vi "IMAQdx_AbsImage_Flea3_v4.6.vi"() -> ()   [LabVIEW 2013] (continued)
  out "Image note":string="Experiment=Sr\nCamera_ID=FL3_32S2M\nImageType=Raw\nDataType=Absorption\nImageDirection=XZ\nMagnification=1.000000E+0\nWMfreq=4.348288461E+2\nLastSave=8a4a9dcffc4e3239d56d97c71c6d4c8385ad02e2\nFileNumber=160\nIndex=0\nIndexedWaves=BBcaptureT;BBcompT;BlueLaserBeatnote;BlueLaserLockOffset;BlueLaserProbeBN;DipAOMFreq;DipPowCr;DipPowCr2;DipPowCr3;DipPowX;DipPowX2;DipPowX3;DipPowX4;DipPowZ;DipPowZ2;DipPowZ3;DipPowZLat;DoppCoolDet;DoppCoolStirDet;DoppCoolSweep;MOTPow;MOTPow2;MOTcurrent;Nspacers;Pdet;PixisPosition;ProbeDet;SFcoolT;TOF;TOFaux;WMfreq;Xshim;Yshim;ZShimVarF;Zshim;ZshimDC;ZshimVar;bLoadT;bMapT;bRampT;combWidthF;combWidthI;depumpOn;depumpPow;dopCoolT;evapOn;freq;holdT;loadT;pulseLatT;rMOTbroadDetuningF;rMOTbroadDetuningI;rMOTcurrF;rMOTcurrI;rMOTon;rMOTpow2;rMOTpow3;rMOTpow4;rMOTpow5;rMOTpow6;rMOTstirDetF;rMOTstirDetI;rampLatOffT;rampLatT;rampOn;rampT;singleFreqDet;singleFreqDetF;singleFreqStirDet;singleFreqStirDetF;tEvap1;tEvap2;tau;tau2;varWaveP1\nIndexedValues=50.0000000000000E-3;400.000000000000E-3;412.000000000000E+3;8.75000000000000E+0;419.000000000000E+3;40.2000000000000E+6;800.000000000000E-3;1.60000000000000E+0;30.0000000000000E-3;1.60000000000000E+0;3.20000000000000E+0;60.0000000000000E-3;30.0000000000000E-3;100.000000000000E-3;400.000000000000E-3;20.0000000000000E-3;150.000000000000E-3;-4.94000000000000E+3;-4.98000000000000E+3;-20.0000000000000E+0;10.0000000000000E+0;2.00000000000000E+0;-6.00000000000000E+0;4.00000000000000E+0;7.00000000000000E+0;15.3000000000000E+0;0.00000000000000E+0;10.0000000000000E-3;11.5000000000000E-3;10.0000000000000E-3;0.00000000000000E+0;230.000000000000E-3;2.55000000000000E+0;1.31500000000000E+0;1.75000000000000E+0;1.31500000000000E+0;1.31500000000000E+0;3.90000000000000E+0;400.000000000000E-6;75.0000000000000E-3;25.0000000000000E-3;2.00000000000000E+0;0.00000000000000E+0;1.00000000000000E+0;25.0000000000000E-3;1.00000000000000E+0;100.000000000000E+0;100.000000000000E-3;45.0000000000000E-3;3.00000000000000E-6;5.56000000000000E+0;5.56000000000000E+0;-290.000000000000E-3;-200.000000000000E-3;1.00000000000000E+0;1.70000000000000E+0;7.10000000000000E+0;1.90000000000000E+0;1.20000000000000E+0;1.65000000000000E+0;6.05000000000000E+0;6.05000000000000E+0;3.00000000000000E-3;50.0000000000000E-3;0.00000000000000E+0;200.000000000000E-3;-5.34000000000000E+3;-5.31000000000000E+3;-5.52000000000000E+3;-5.45000000000000E+3;3.20000000000000E+0;3.50000000000000E+0;1.00000000000000E+0;6.00000000000000E+0;2.65000000000000E+0\n# Current Variables\n#\nZShimVarF = 1.315000E+0\nZshimVar = 1.315000E+0\nBBcaptureT = 5.000000E-2\nBBcompT = 4.000000E-1\nBlueDipPow = 2.400000E-1\nBlueLaserBeatnote = 4.120000E+5\nBlueLaserLockOffset = 8.750000E+0\nBlueLaserProbeBN = 4.190000E+5\nDipAOMFreq = 4.020000E+7\nDipPowCr = 8.000000E-1\nDipPowCr2 = 1.600000E+0\nDipPowCr3 = 3.000000E-2\nDipPowCr4 = 1.500000E-2\nDipPowCrTOF = 8.000000E-1\nDipPowHLat = 7.700000E-2\nDipPowHLat2 = 4.500000E-1\nDipPowX = 1.600000E+0\nDipPowX2 = 3.200000E+0\nDipPowX3 = 6.000000E-2\nDipPowX4 = 3.000000E-2\nDipPowXLat = 1.000000E+0\nDipPowXTOF = 1.600000E+0\nDipPowZ = 1.000000E-1\nDipPowZ2 = 4.000000E-1\nDipPowZ3 = 2.000000E-2\nDipPowZ4 = 1.000000E-2\nDipPowZLat = 1.500000E-1\nDoppCoolDet = -4.940000E+3\nDoppCoolPow = 1.250000E+0\nDoppCoolStirDet = -4.980000E+3\nDoppCoolSweep = -2.000000E+1\nDoppStirPow = 1.600000E+0\nHeatingAmp = 1.000000E-1\nHimaging = 1.000000E+0\nMOTPow = 1.000000E+1\nMOTPow2 = 2.000000E+0\nMOTcurrent = -6.000000E+0\nMOTcurrent2 = -7.500000E+0\nMOTdetuning = -4.504000E+1\nNspacers = 4.000000E+0\nPdet = 7.000000E+0\nPdet2 = 5.000000E-2\nPixisPosition = 1.530000E+1\nProbeDet = 0.000000E+0\nProbePow = 1.420000E+0\nSFcoolT = 1.000000E-2\nTOF = 1.150000E-2\nTOFaux = 1.000000E-2\nVimaging = 1.000000E+0\nWMfreq = 0.000000E+0\nXshim = 2.300000E-1\nXshimDC = 2.500000E-1\nYshim = 2.550000E+0\nYshimDC = 2.575000E+0\nZshim = 1.750000E+0\nZshimDC = 1.315000E+0\nbLoadT = 3.900000E+0\nbMOToverride = 1.000000E+0\nbMapT = 4.000000E-4\nbRampT = 7.500000E-2\ncameraArmT = 1.500000E-3\ncombWidthF = 2.500000E-2\ncombWidthI = 2.000000E+0\ncompensation = -3.981000E+0\ndepumpOn = 0.000000E+0\ndepumpPow = 1.000000E+0\ndopCoolT = 2.500000E-2\ndopCoolT1 = 5.000000E-3\nevapOn = 1.000000E+0\nexposureT = 1.000000E-5\nfreq = 1.000000E+2\nholdT = 1.000000E-1\nloadT = 4.500000E-2\nminus_zman = -7.904000E+0\nplus_zman = -9.792000E+0\npulseLatT = 3.000000E-6\nrMOTbroadDetuningF = 5.560000E+0\nrMOTbroadDetuningI = 5.560000E+0\nrMOTcurrF = -2.900000E-1\nrMOTcurrI = -2.000000E-1\nrMOTon = 1.000000E+0\nrMOTpow1 = 7.000000E+0\nrMOTpow2 = 1.700000E+0\nrMOTpow3 = 7.100000E+0\nrMOTpow4 = 1.900000E+0\nrMOTpow5 = 1.200000E+0\nrMOTpow6 = 1.650000E+0\nrMOTstirDetF = 6.050000E+0\nrMOTstirDetI = 6.050000E+0\nrampLatOffT = 3.000000E-3\nrampLatT = 5.000000E-2\nrampOn = 0.000000E+0\nrampT = 2.000000E-1\nsingleFreqDet = -5.340000E+3\nsingleFreqDetF = -5.310000E+3\nsingleFreqStirDet = -5.520000E+3\nsingleFreqStirDetF = -5.450000E+3\nstirWidthF = 2.500000E-2\nstirWidthI = 2.000000E+0\ntEvap0 = 1.000000E-1\ntEvap1 = 3.200000E+0\ntEvap2 = 3.500000E+0\ntau = 1.000000E+0\ntau2 = 6.000000E+0\nvarWaveP1 = 2.650000E+0\nvarWaveP2 = 1.200000E+0\n#\n# Master Staging List\n#Comment\tMarker\tMode\tGroup\tDelay\tX ODT Shuttter\tX ODT AO TTL\tVert ODT Shutter\tVert ODT AO TTL\tCross ODT Shutter\tCross ODT AO TTL\t707 Shutter\tPB_7\tH Probe AO TTL\tFreq Switch rMOT\trMOT AO TTL\t\tTrans AO TTL\tV Probe AO TTL\tZman AO TTL\tbMOT AO TTL\t60 Hz Trig Gate\tWindow Heater TTL\tPB_18\t\tPB_20 Trigger Dev3\tPB_21 Trigger Dev2\tPB_22 Trigger Dev1\tPB_23 Trigger Dev0\tStep\t~Atomic Beam Shutter\tGate Valve\tDO0_2\t707b Shutter\t~Zman Coils\t~ MOT Coils\t~ Dipole Flea3 Shutter\trMOT Shutter\t+Zeeman Coils\t-Zeeman Coils\tCompensation Coils\tMOT Coils\trMOT AO Power\trMOT Freq Amplitude\trMOT Freq Offset\tH Lattice AO Power\tTrans Shutter\tV Probe Shutter\tZman Shutter\tbMOT Shutter\tDO1_4\t679 Shutter\t~Pixis Shutter\t~Abs Flea3 Shutter\tAO1_0\tMOT AO Power\tProbe AO Power\tAO1_3\tX Shim Coils\tY Shim Coils\tZ Shim Coils\tVert ODT AO Power\tPIXIS Ext Shutter\tBlueODT TTL\tBlueODT Shutter\tH Probe Shutter\tH Lattice Shutter\tH Lattice AO TTL\tParametric Heating\t689c AOM TTL\tAO2_0\tAO2_1\tD03_0\tD03_1\tD03_2\tD03_3\tD03_4\tD03_5\tD03_6\tD03_7\trMOT Stir Freq Offset\tBlueODT Power\tCrossODT Power\tVariable Waveplate\tAO3_4\tAO3_5\trMOT Stir Power\tX ODT AO Power\tSRS Freq\tSRS Amp\tSRS Offset\tSRS Func Type\tRedMotDDS\tRedMotDDS_ 0\tRedMotDDS_ 1\tRedMotDDS_ 2\tStirringDDS\tStirringDDS_ 0\tStirringDDS_ 1\tStirringDDS_ 2\tBlueBN\tBlueBN_ 0\tPosition\tRun Mode\r\n\r\nreset\t\tRamp\t1\t.1\t1\t1\t1\t1\t1\t1\t1\t0\t1\t0\t1\t0\t1\t1\t1\t0\t0\t0\t0\t0\t0\t0\t0\t0\t0\t0\t1\t0\t1\t0\t0\t1\t0\tplus_zman\tminus_zman\tcompensation\tMOTcurrent\trMOTpow1\tcombAmplitude(combWidthI)\trMOTdelta(-(rMOTbroadDetuningI +combWidthI/2))\tODTpowHLat(DipPowHLat2)\t0\t0\t1\t0\t0\t1\t1\t1\tbMOTdelta(MOTdetuning)\tbMOTpow(0.5)\tProbePow\tPdet2\tXshim\tYshim\tZshim\tODTpowZ(DipPowZ)\t0\t1\t0\t0\t0\t1\t0\t0\t0\t0\t0\t0\t0\t0\t0\t0\t0\t0\trMOTdelta(-(rMOTstirDetI +stirWidthI/2))\tODTpowBlue(0)\tODTpowXY(DipPowCr)\tvarWaveP1\tBlueLaserLockOffset\tAmp688(depumpPow)\trMOTpow3\tODTpowX(DipPowX)\tfreq\tHeatingAmp\t0\tSine\tDetuning\tsingleFreqDet\t-20\t8\tDetuning\tsingleFreqStirDet\t0\t0\tBlueBN\tBlueLaserBeatnote\tPixisPos(TOF)\tCycle Wait for Move\r\nblue MOT load\t\tRamp\t0\tbLoadT\t1\t1\t1\t1\t1\t1\t1\t0\t1\t0\t1\t0\t1\t1\t1\t1\t0\t0\t0\t0\t0\t0\t0\t0\t0\t0\t1\t0\t1\t0\t0\t1\t1\tplus_zman\tminus_zman\tcompensation\tMOTcurrent\trMOTpow1\tcombAmplitude(combWidthI)\trMOTdelta(-(rMOTbroadDetuningI +combWidthI/2))\tODTpowHLat(DipPowHLat)\t1\t0\t1\tbMOToverride\t1\t1\t1\t1\tbMOTdelta(MOTdetuning)\tbMOTpow(MOTPow)\tProbePow\tPdet2\tXshim\tYshim\tZshim\tODTpowZ(DipPowZ)\t0\t1\t0\t0\t0\t1\t0\t0\t0\t0\t0\t0\t0\t0\t0\t0\t0\t0\trMOTdelta(-(rMOTstirDetI +stirWidthI/2))\tODTpowBlue(0)\tODTpowXY(DipPowCr)\tvarWaveP1\tBlueLaserLockOffset\tAmp688(depumpPow)\trMOTpow3\tODTpowX(DipPowX)\tfreq\tHeatingAmp\t0\tSine\tDetuning\tsingleFreqDet\t-20\t8\tDetuning\tsingleFreqStirDet\t0\t0\tBlueBN\tBlueLaserBeatnote\tPixisPos(TOF)\tCycle Wait for Move\r\npretrig\t\tRamp\t1\t500m\t1\t1\t1\t1\t1\t0\t1\t0\t1\t0\t1\t0\t1\t1\t1\t1\t0\t1\t0\t0\t0\t0\t0\t0\t0\t0\t1\t0\t1\t0\t0\t0\t1\tplus_zman\tminus_zman\tcompensation\tMOTcurrent\trMOTpow1\tcombAmplitude(combWidthI)\trMOTdelta(-(rMOTbroadDetuningI +combWidthI/2))\tODTpowHLat(DipPowHLat2)\t1\t0\t1\tbMOToverride\t1\t1\t0\t0\tbMOTdelta(MOTdetuning)\tbMOTpow(MOTPow)\tProbePow\tPdet2\tXshim\tYshim\tZshim\tODTpowZ(DipPowZ)\t0\t1\t0\t0\t1\t1\t0\t0\t0\t0\t0\t0\t0\t0\t0\t0\t0\t0\trMOTdelta(-(rMOTstirDetI +stirWidthI/2))\tODTpowBlue(0)\tODTpowXY(DipPowCr)\tvarWaveP1\tBlueLaserLockOffset\tAmp688(depumpPow)\trMOTpow3\tODTpowX(DipPowX)\tfreq\tHeatingAmp\t0\tSine\tDetuning\tsingleFreqDet\t-20\t8\tDetuning\tsingleFreqStirDet\t0\t0\tBlueBN\tBlueLaserBeatnote\tPixisPos(TOF)\tCycle Wait for Move\r\nblue MOT load\t\tRamp\t1\tbLoadT\t1\t1\t1\t1\t1\t1\t1\t0\t1\t0\t1\t0\t1\t1\t1\t1\t0\t0\t0\t0\t0\t0\t0\t0\t0\t0\t1\t0\t1\t0\t0\t1\t1\tplus_zman\tminus_zman\tcompensation\tMOTcurrent\trMOTpow1\tcombAmplitude(combWidthI)\trMOTdelta(-(rMOTbroadDetuningI +combWidthI/2))\tODTpowHLat(DipPowHLat)\t1\t0\t1\tbMOToverride\t1\t1\t1\t1\tbMOTdelta(MOTdetuning)\tbMOTpow(MOTPow)\tProbePow\tPdet2\tXshim\tYshim\tZshim\tODTpowZ(DipPowZ)\t0\t1\t0\t0\t0\t1\t0\t0\t0\t0\t0\t0\t0\t0\t0\t0\t0\t0\trMOTdelta(-(rMOTstirDetI +stirWidthI/2))\tODTpowBlue(0)\tODTpowXY(DipPowCr)\tvarWaveP1\tBlueLaserLockOffset\tAmp688(depumpPow)\trMOTpow3\tODTpowX(DipPowX)\tfreq\tHeatingAmp\t0\tSine\tDetuning\tsingleFreqDet\t-20\t8\tDetuning\tsingleFreqStirDet\t0\t0\tBlueBN\tBlueLaserBeatnote\tPixisPos(TOF)\tCycle Wait for Move\r\ndump bMOT\t\tRamp\t1\t0.1-bRampT\t1\t1\t1\t1\t1\t1\t1\t0\t1\t0\t1\t0\t1\t1\t1\t1\t0\t1\t0\t0\t0\t0\t0\t0\t1m\t0\t1\t0\t1\t0\t0\t1\t1\tplus_zman\tminus_zman\tcompensation\tMOTcurrent\trMOTpow1\tcombAmplitude(combWidthI)\trMOTdelta(-(rMOTbroadDetuningI +combWidthI/2))\tODTpowHLat(DipPowHLat)\t1\t0\t1\tbMOToverride\t1\t1\t1\t1\tbMOTdelta(MOTdetuning)\tbMOTpow(MOTPow)\tProbePow\tPdet2\tXshim\tYshim\tZshim\tODTpowZ(DipPowZ)\t0\t1\t0\t0\t0\t1\t0\t0\t0\t0\t0\t0\t0\t0\t0\t0\t0\t0\trMOTdelta(-(rMOTstirDetI +stirWidthI/2))\tODTpowBlue(0)\tODTpowXY(DipPowCr)\tvarWaveP1\tBlueLaserLockOffset\tAmp688(depumpPow)\trMOTpow3\tODTpowX(DipPowX)\tfreq\tHeatingAmp\t0\tSine\tDetuning\tsingleFreqDet\t-20\t8\tDetuning\tsingleFreqStirDet\t0\t0\tBlueBN\tBlueLaserBeatnote\tPixisPos(TOF)\tCycle Wait for Move\r\ndump bMOT\t\tRamp\t1\tbRampT\t1\t1\t1\t1\t1\t1\t1\t0\t1\t0\t1\t0\t1\t1\t1\t1\t0\t1\t0\t0\t0\t0\t0\t0\t1m\t0\t1\t0\t1\t0\t0\t1\t1\tplus_zman\tminus_zman\tcompensation\tLineRamp(f,MOTcurrent,MOTcurrent2)\trMOTpow1\tcombAmplitude(combWidthI)\trMOTdelta(-(rMOTbroadDetuningI +combWidthI/2))\tODTpowHLat(DipPowHLat)\t1\t0\t1\tbMOToverride\t1\t1\t1\t1\tbMOTdelta(MOTdetuning)\tLineRamp(f,bMOTpow(MOTPow),bMOTpow(MOTPow2))\tProbePow\tPdet2\tXshim\tYshim\tZshim\tODTpowZ(DipPowZ)\t0\t1\t0\t0\t0\t1\t0\t0\t0\t0\t0\t0\t0\t0\t0\t0\t0\t0\trMOTdelta(-(rMOTstirDetI +stirWidthI/2))\tODTpowBlue(0)\tODTpowXY(DipPowCr)\tvarWaveP1\tBlueLaserLockOffset\tAmp688(depumpPow)\trMOTpow3\tODTpowX(DipPowX)\tfreq\tHeatingAmp\t0\tSine\tDetuning\tsingleFreqDet\t-20\t8\tDetuning\tsingleFreqStirDet\t0\t0\tBlueBN\tBlueLaserBeatnote\tPixisPos(TOF)\tCycle Wait for Move\r\nCamWaitTime\t\tRamp\t0\t.1\t1\t1\t1\t1\t1\t1\t1\t0\t0\t0\t1\t0\t1\t0\t1\t1\t0\t1\t0\t0\t0\t0\t0\t0\t0\t0\t1\t0\t1\t0\t0\t1\t1\tplus_zman\tminus_zman\tcompensation\tMOTcurrent\trMOTpow1\tcombAmplitude(combWidthI)\trMOTdelta(-(rMOTbroadDetuningI +combWidthI/2))\tODTpowHLat(DipPowHLat)\t1\t0\t1\tbMOToverride\t1\t1\t1\t1\tbMOTdelta(MOTdetuning)\tbMOTpow(MOTPow2)\tProbePow\tPdet2\tXshim\tYshim\tZshim\tODTpowZ(DipPowZ)\t0\t1\t0\t0\t0\t1\t0\t0\t0\t0\t0\t0\t0\t0\t0\t0\t0\t0\trMOTdelta(-(rMOTstirDetI +stirWidthI/2))\tODTpowBlue(0)\tODTpowXY(DipPowCr)\tvarWaveP1\tBlueLaserLockOffset\tAmp688(depumpPow)\trMOTpow3\tODTpowX(DipPowX)\tfreq\tHeatingAmp\t0\tSine\tDetuning\tsingleFreqDet\t-20\t8\tDetuning\tsingleFreqStirDet\t0\t0\tBlueBN\tBlueLaserBeatnote\tPixisPos(TOF)\tCycle Wait for Move\r\nProbeShutOn\t\tRamp\t1-rMOTon\t1120e-6\t1\t1\t1\t1\t1\t1\t1\t0\t0\t0\t1\t0\t0\t0\t0\t1\t0\t1\t0\t0\t0\t0\t0\t0\t0\t0\t1\t0\t1\t0\t0\t1\t1\tplus_zman\tminus_zman\tcompensation\tMOTcurrent\trMOTpow1\tcombAmplitude(combWidthI)\trMOTdelta(-(rMOTbroadDetuningI +combWidthI/2))\tODTpowHLat(DipPowHLat)\t1\t0\t1\tbMOToverride\t1\t1\t1\t1\tbMOTdelta(MOTdetuning)\tbMOTpow(MOTPow2)\tProbePow\tPdet2\tXshim\tYshim\tZshim\tODTpowZ(DipPowZ)\t0\t1\t0\tHimaging\t0\t1\t0\t0\t0\t0\t0\t0\t0\t0\t0\t0\t0\t0\trMOTdelta(-(rMOTstirDetI +stirWidthI/2))\tODTpowBlue(0)\tODTpowXY(DipPowCr)\tvarWaveP1\tBlueLaserLockOffset\tAmp688(depumpPow)\trMOTpow3\tODTpowX(DipPowX)\tfreq\tHeatingAmp\t0\tSine\tDetuning\tsingleFreqDet\t-20\t8\tDetuning\tsingleFreqStirDet\t0\t0\tBlueBN\tBlueLaserBeatnote\tPixisPos(TOF)\tCycle Wait for Move\r\nRepumpShutOff\t\tRamp\t1-rMOTon\t260e-6\t1\t1\t1\t1\t1\t1\t1\t0\t0\t0\t1\t0\t0\t0\t0\t1\t0\t1\t0\t0\t0\t0\t0\t0\t0\t0\t1\t0\t1\t0\t0\t1\t1\tplus_zman\tminus_zman\tcompensation\tMOTcurrent\trMOTpow1\tcombAmplitude(combWidthI)\trMOTdelta(-(rMOTbroadDetuningI +combWidthI/2))\tODTpowHLat(DipPowHLat)\t1\t0\t0\tbMOToverride\t1\t1\t1\t1\tbMOTdelta(MOTdetuning)\tbMOTpow(MOTPow2)\tProbePow\tPdet2\tXshim\tYshim\tZshim\tODTpowZ(DipPowZ)\t0\t1\t0\tHimaging\t0\t1\t0\t0\t0\t0\t0\t0\t0\t0\t0\t0\t0\t0\trMOTdelta(-(rMOTstirDetI +stirWidthI/2))\tODTpowBlue(0)\tODTpowXY(DipPowCr)\tvarWaveP1\tBlueLaserLockOffset\tAmp688(depumpPow)\trMOTpow3\tODTpowX(DipPowX)\tfreq\tHeatingAmp\t0\tSine\tDetuning\tsingleFreqDet\t-20\t8\tDetuning\tsingleFreqStirDet\t0\t0\tBlueBN\tBlueLaserBeatnote\tPixisPos(TOF)\tCycle Wait for Move\r\nMOTShutOff\t\tRamp\t1-rMOTon\t1370e-6\t1\t1\t1\t1\t1\t1\t1\t0\t0\t0\t1\t0\t0\t0\t0\t1\t0\t1\t0\t0\t0\t0\t0\t0\t0\t0\t1\t0\t1\t0\t0\t1\t1\tplus_zman\tminus_zman\tcompensation\tMOTcurrent\trMOTpow1\tcombAmplitude(combWidthI)\trMOTdelta(-(rMOTbroadDetuningI +combWidthI/2))\tODTpowHLat(DipPowHLat)\t1\t0\t0\t0\t1\t1\t1\t1\tbMOTdelta(MOTdetuning)\tbMOTpow(MOTPow2)\tProbePow\tPdet2\tXshim\tYshim\tZshim\tODTpowZ(DipPowZ)\t0\t1\t0\tHimaging\t0\t1\t0\t0\t0\t0\t0\t0\t0\t0\t0\t0\t0\t0\trMOTdelta(-(rMOTstirDetI +stirWidthI/2))\tODTpowBlue(0)\tODTpowXY(DipPowCr)\tvarWaveP1\tBlueLaserLockOffset\tAmp688(depumpPow)\trMOTpow3\tODTpowX(DipPowX)\tfreq\tHeatingAmp\t0\tSine\tDetuning\tsingleFreqDet\t-20\t8\tDetuning\tsingleFreqStirDet\t0\t0\tBlueBN\tBlueLaserBeatnote\tPixisPos(TOF)\tCycle Wait for Move\r\nCoil Switch\t\tRamp\trMOTon\t220e-6\t1\t1\t1\t1\t1\t1\t1\t0\t1\t0\t1\t0\t0\t1\t0\t1\t0\t1\t0\t0\t0\t0\t0\t0\t0\t0\t1\t0\t1\t0\t0\t1\t1\tplus_zman\tminus_zman\tcompensation\trMOTcurrI\trMOTpow1\tcombAmplitude(combWidthI)\trMOTdelta(-(rMOTbroadDetuningI +combWidthI/2))\tODTpowHLat(DipPowHLat)\t1\t0\t0\t0\t1\t1\t1\t1\tbMOTdelta(MOTdetuning)\tbMOTpow(2)\tProbePow\tPdet2\tXshim\tYshim\tZshim\tODTpowZ(DipPowZ)\t0\t1\t0\t0\t0\t1\t0\t0\t0\t0\t0\t0\t0\t0\t0\t0\t0\t0\trMOTdelta(-(rMOTstirDetI +stirWidthI/2))\tODTpowBlue(0)\tODTpowXY(DipPowCr)\tvarWaveP1\tBlueLaserLockOffset\tAmp688(depumpPow)\trMOTpow3\tODTpowX(DipPowX)\tfreq\tHeatingAmp\t0\tSine\tDetuning\tsingleFreqDet\t-20\t8\tDetuning\tsingleFreqStirDet\t0\t0\tBlueBN\tBlueLaserBeatnote\tPixisPos(TOF)\tCycle Wait for Move\r\n60HzTrigger\t\tHalt\t0\t10u\t1\t1\t1\t1\t1\t1\t1\t0\t0\t0\t1\t0\t0\t0\t0\t0\t0\t1\t0\t0\t0\t0\t0\t0\t0\t0\t1\t0\t1\t0\t0\t1\t1\tplus_zman\tminus_zman\tcompensation\trMOTcurrI\trMOTpow1\tcombAmplitude(combWidthI)\trMOTdelta(-(rMOTbroadDetuningI +combWidthI/2))\tODTpowHLat(DipPowHLat)\t1\t0\t0\t0\t1\t1\t1\t1\tbMOTdelta(MOTdetuning)\tbMOTpow(2)\tProbePow\tPdet2\tXshim\tYshim\tZshim\tODTpowZ(DipPowZ)\t0\t1\t0\t0\t0\t1\t0\t0\t0\t0\t0\t0\t0\t0\t0\t0\t0\t0\trMOTdelta(-(rMOTstirDetI +stirWidthI/2))\tODTpowBlue(0)\tODTpowXY(DipPowCr)\tvarWaveP1\tBlueLaserLockOffset\tAmp688(depumpPow)\trMOTpow3\tODTpowX(DipPowX)\tfreq\tHeatingAmp\t0\tSine\tDetuning\tsingleFreqDet\t-20\t8\tDetuning\tsingleFreqStirDet\t0\t0\tBlueBN\tBlueLaserBeatnote\tPixisPos(TOF)\tCycle Wait for Move\r\nCapture Red MOT\t\tRamp\trMOTon\tBBcaptureT\t1\t1\t1\t1\t1\t1\t1\t0\t1\t0\t1\t0\t0\t1\t0\t0\t0\t1\t0\t0\t0\t0\t0\t0\t1m\t0\t1\t0\t1\t0\t0\t1\t1\tplus_zman\tminus_zman\tcompensation\trMOTcurrI\trMOTpow1\tcombAmplitude(combWidthI)\trMOTdelta(-(rMOTbroadDetuningI +combWidthI/2))\tODTpowHLat(DipPowHLat)\t0\t0\t0\t0\t1\t1\t1\t1\tbMOTdelta(MOTdetuning)\tbMOTpow(0.5)\tProbePow\tPdet2\tXshim\tYshim\tZshim\tODTpowZ(DipPowZ)\t0\t1\t0\t0\t0\t1\t0\t0\t0\t0\t0\t0\t0\t0\t0\t0\t0\t0\trMOTdelta(-(rMOTstirDetI +stirWidthI/2))\tODTpowBlue(0)\tODTpowXY(DipPowCr)\tvarWaveP1\tBlueLaserLockOffset\tAmp688(depumpPow)\trMOTpow3\tODTpowX(DipPowX)\tfreq\tHeatingAmp\t0\tSine\tDetuning\tsingleFreqDet\t-20\t8\tDetuning\tsingleFreqStirDet\t0\t0\tBlueBN\tBlueLaserProbeBN\tPixisPos(TOF)\tCycle Wait for Move\r\nRamp Red MOT\t\tRamp\trMOTon\tBBcompT\t1\t1\t1\t1\t1\t1\t1\t0\t1\t0\t1\t0\t0\t1\t0\t0\t0\t1\t0\t0\t0\t0\t0\t0\t10u\t0\t1\t0\t1\t0\t0\t1\t1\tplus_zman\tminus_zman\tcompensation\tLineRamp(f,rMOTcurrI,rMOTcurrF)\tHalfGaussRamp(t,rMOTpow1,rMOTpow2, BBcompT)\tLineRamp(f,combAmplitude(combWidthI),combAmplitude(combWidthF))\tLineRamp(f,rMOTdelta(-(rMOTbroadDetuningI +combWidthI/2)),rMOTdelta(-(rMOTbroadDetuningF +combWidthF/2)))\tODTpowHLat(DipPowHLat)\t0\t0\t0\t0\t1\t1\t1\t1\tbMOTdelta(MOTdetuning)\tbMOTpow(0.5)\tProbePow\tPdet2\tXshim\tYshim\tLineRamp(f,Zshim,ZshimVar)\tODTpowZ(DipPowZ)\t0\t1\t0\t0\t0\t1\t0\t0\t0\t0\t0\t0\t0\t0\t0\t0\t0\t0\tLineRamp(f,rMOTdelta(-(rMOTstirDetI +stirWidthI/2)),rMOTdelta(-(rMOTstirDetF +stirWidthF/2)))\tODTpowBlue(0)\tODTpowXY(DipPowCr)\tvarWaveP1\tLineRamp(f,BlueLaserLockOffset,Pdet)\tAmp688(depumpPow)\tHalfGaussRamp(t,rMOTpow3,rMOTpow4, BBcompT)\tODTpowX(DipPowX)\tfreq\tHeatingAmp\t0\tSine\tDetuning\tsingleFreqDet\t-20\t8\tDetuning\tsingleFreqStirDet\t0\t0\tBlueBN\tBlueLaserProbeBN\tPixisPos(TOF)\tCycle Wait for Move\r\nBB load\t\tRamp\t0\tloadT\t1\t1\t1\t1\t1\t1\t0\t0\t0\t0\t1\t0\t0\t0\t0\t0\t0\t1\t0\t0\t0\t0\t0\t0\t10u\t0\t1\t0\t0\t0\t0\t1\t1\tplus_zman\tminus_zman\tcompensation\trMOTcurrF\trMOTpow2\tcombAmplitude(combWidthF)\trMOTdelta(-(rMOTbroadDetuningF +combWidthF/2))\tODTpowHLat(DipPowHLat)\t0\t0\t0\t0\t1\t0\t1\t1\tbMOTdelta(MOTdetuning)\tbMOTpow(0.5)\tProbePow\tPdet2\tXshim\tYshim\tLineRamp(f,ZshimVar,ZShimVarF)\tODTpowZ(DipPowZ)\t0\t1\t0\t0\t0\t1\t0\t0\t0\t0\t0\t0\t0\t0\t0\t0\t0\t0\trMOTdelta(-(rMOTstirDetF +stirWidthF/2))\tODTpowBlue(0)\tODTpowXY(DipPowCr)\tvarWaveP1\tPdet\tAmp688(depumpPow)\trMOTpow4\tODTpowX(DipPowX)\tfreq\tHeatingAmp\t0\tSine\tDetuning\tsingleFreqDet\t-20\t8\tDetuning\tsingleFreqStirDet\t0\t0\tBlueBN\tBlueLaserProbeBN\tPixisPos(TOF)\tCycle Wait for Move\r\nSF\t\tRamp\t1\tSFcoolT\t1\t1\t1\t1\t1\t1\t0\t0\t0\t1\t1\t0\t0\t0\t0\t0\t0\t1\t0\t0\t0\t0\t0\t0\t10u\t0\t1\t0\t0\t0\t0\t1\t1\tplus_zman\tminus_zman\tcompensation\trMOTcurrF\trMOTpow2\tcombAmplitude(combWidthF)\trMOTdelta(-(rMOTbroadDetuningF +combWidthF/2))\tODTpowHLat(DipPowHLat)\t0\t0\t0\t0\t1\t0\t1\t1\tbMOTdelta(MOTdetuning)\tbMOTpow(0.5)\tProbePow\tPdet2\tXshim\tYshim\tZshimVar\tODTpowZ(DipPowZ)\t0\t1\t0\t0\t0\t1\t0\t0\t0\t0\t0\t0\t0\t0\t0\t0\t0\t0\trMOTdelta(-(rMOTstirDetF +stirWidthF/2))\tODTpowBlue(0)\tODTpowXY(DipPowCr)\tvarWaveP1\tPdet\tAmp688(depumpPow)\trMOTpow4\tODTpowX(DipPowX)\tfreq\tHeatingAmp\t0\tSine\tRamp\tsingleFreqDet\tsingleFreqDet + 20\tSFCoolT*1000\tRamp\tsingleFreqStirDet\tsingleFreqStirDet + 20\tSFcoolT*1000\tBlueBN\tBlueLaserProbeBN\tPixisPos(TOF)\tCycle Wait for Move\r\nload1\t\tRamp\t1\tloadT\t1\t1\t1\t1\t1\t1\t1\t0\t1\t1\t1\t0\t0\t1\t0\t0\t0\t1\t0\t0\t0\t0\t0\t0\t10u\t0\t1\t0\t0\t0\t0\t1\t1\tplus_zman\tminus_zman\tcompensation\trMOTcurrF\tLineRamp(f,rMOTpow2,rMOTpow5)\tcombAmplitude(combWidthF)\trMOTdelta(-(rMOTbroadDetuningF +combWidthF/2))\tODTpowHLat(DipPowHLat)\t0\t0\t0\t0\t1\t0\t1\t1\tbMOTdelta(MOTdetuning)\tbMOTpow(0.5)\tProbePow\tPdet2\tXshim\tYshim\tLineRamp(f,ZshimVar,ZShimVarF)\tODTpowZ(DipPowZ)\t0\t1\t0\t0\t0\t1\t0\t0\t0\t0\t0\t0\t0\t0\t0\t0\t0\t0\trMOTdelta(-(rMOTstirDetF +stirWidthF/2))\tODTpowBlue(0)\tODTpowXY(DipPowCr)\tvarWaveP1\tPdet\tAmp688(depumpPow)\tLineRamp(f,rMOTpow4,rMOTpow6)\tODTpowX(DipPowX)\tfreq\tHeatingAmp\t0\tSine\tDetuning\tsingleFreqDetF\tsingleFreqDet + 20\tSFCoolT*1000\tDetuning\tsingleFreqStirDet + 20\tsingleFreqStirDet + 20\tSFcoolT*1000\tBlueBN\tBlueLaserProbeBN\tPixisPos(TOF)\tCycle Wait for Move\r\nload2\t\tRamp\t0\t.05\t1\t1\t1\t1\t1\t1\t0\t0\t1\t1\t1\t0\t0\t1\t0\t0\t0\t1\t0\t0\t0\t0\t0\t0\t0\t0\t1\t0\t0\t0\t0\t1\t1\tplus_zman\tminus_zman\tcompensation\trMOTcurrF\trMOTpow5\tcombAmplitude(combWidthF)\trMOTdelta(-(rMOTbroadDetuningF +combWidthF/2))\tODTpowHLat(DipPowHLat)\t0\t0\t0\t0\t1\t0\t1\t1\tbMOTdelta(MOTdetuning)\tbMOTpow(0.5)\tProbePow\tPdet2\tXshim\tYshim\tZshimVar\tODTpowZ(DipPowZ)\t0\t1\t0\t0\t0\t1\t0\t0\t0\t0\t0\t0\t0\t0\t0\t0\t0\t0\trMOTdelta(-(rMOTstirDetF +stirWidthF/2))\tODTpowBlue(0)\tODTpowXY(DipPowCr)\tvarWaveP1\tPdet\tAmp688(depumpPow)\trMOTpow6\tODTpowX(DipPowX)\tfreq\tHeatingAmp\t0\tSine\tDetuning\tsingleFreqDetF\tsingleFreqDet + 20\tSFCoolT*1000\tDetuning\tsingleFreqStirDetF\tsingleFreqStirDet + 20\tSFcoolT*1000\tBlueBN\tBlueLaserProbeBN\tPixisPos(TOF)\tCycle Wait for Move\r\ndrop Red MOT\t\tRamp\t0\t.15\t1\t1\t0\t0\t0\t0\t0\t0\t1\t1\t0\t0\t0\t1\t0\t0\t0\t1\t0\t0\t0\t0\t0\t0\t0\t0\t1\t0\t0\t0\t1\t1\t0\tplus_zman\tminus_zman\tcompensation\trMOTcurrF\trMOTpow5\tcombAmplitude(combWidthF)\trMOTdelta(-(rMOTbroadDetuningF +combWidthF/2))\tODTpowHLat(DipPowHLat2)\t0\t0\t0\t0\t0\t0\t1\t1\tbMOTdelta(MOTdetuning)\tbMOTpow(0.5)\tProbePow\tPdet2\tXshim\tYshim\tZShimVarF\tODTpowZ(DipPowZ)\t0\t1\t0\t0\t1\t1\t0\t0\t0\t0\t0\t0\t0\t0\t0\t0\t0\t0\trMOTdelta(-(rMOTstirDetF +stirWidthF/2))\tODTpowBlue(0)\tODTpowXY(DipPowCr)\tvarWaveP1\tPdet\tAmp688(depumpPow)\trMOTpow6\tODTpowX(DipPowX)\tfreq\tHeatingAmp\t0\tSine\tDetuning\tDoppCoolDet\tsingleFreqDet + 20\tSFCoolT*1000\tDetuning\tDoppCoolStirDet\tsingleFreqStirDet + 20\tSFcoolT*1000\tBlueBN\tBlueLaserProbeBN\tPixisPos(TOF)\tCycle Wait for Move\r\nramp Trap\t\tRamp\t1\trampT\t1\t1\t1\t1\t1\t1\t0\t0\t1\t1\t0\t0\t0\t1\t0\t0\t0\t1\t0\t0\t0\t0\t0\t0\t10u\t0\t1\t0\t0\t0\t1\t1\t0\tplus_zman\tminus_zman\tcompensation\trMOTcurrF\trMOTpow3\tcombAmplitude(combWidthF)\trMOTdelta(-(rMOTbroadDetuningF +combWidthF/2))\tODTpowHLat(DipPowHLat)\t0\t0\t0\t0\t0\t0\t1\t1\tbMOTdelta(MOTdetuning)\tbMOTpow(0.5)\tProbePow\tPdet2\tXshimDC\tYshimDC\tZshimDC\tSinRamp(t,(ODTpowZ(DipPowZ)+ODTpowZ(DipPowZ2))/2,(ODTpowZ(DipPowZ2)-ODTpowZ(DipPowZ))/2,1/(2*rampT),3*pi/2)\t0\t1\t0\t0\t0\t1\t0\t0\t0\t0\t0\t0\t0\t0\t0\t0\t0\t0\trMOTdelta(-(rMOTstirDetI +stirWidthF/2))\tODTpowBlue(0)\tSinRamp(t,(ODTpowXY(DipPowCr)+ODTpowXY(DipPowCr2))/2,(ODTpowXY(DipPowCr2)-ODTpowXY(DipPowCr))/2,1/(2*rampT),3*pi/2)\tvarWaveP1\tPdet\tAmp688(depumpPow)\trMOTpow6\tSinRamp(t,(ODTpowX(DipPowX)+ODTpowX(DipPowX2))/2,(ODTpowX(DipPowX2)-ODTpowX(DipPowX))/2,1/(2*rampT),3*pi/2)\tfreq\tHeatingAmp\t0\tSine\tDetuning\tsingleFreqDetF\tsingleFreqDet + 20\tSFCoolT*1000\tDetuning\tsingleFreqStirDetF\tsingleFreqStirDet + 20\tSFcoolT*1000\tBlueBN\tBlueLaserProbeBN\tPixisPos(TOF)\tCycle Wait for Move\r\nhold\t\tRamp\t0\t.01\t1\t1\t1\t1\t1\t1\t0\t0\t1\t1\t0\t0\t0\t1\t0\t0\t0\t1\t0\t0\t0\t0\t0\t0\t0\t0\t1\t0\t0\t0\t1\t1\t0\tplus_zman\tminus_zman\tcompensation\trMOTcurrF\trMOTpow4\tcombAmplitude(combWidthF)\trMOTdelta(-(rMOTbroadDetuningF +combWidthF/2))\tODTpowHLat(DipPowHLat)\t0\t0\t0\t0\t1\t0\t1\t1\tbMOTdelta(MOTdetuning)\tbMOTpow(0.5)\tProbePow\tPdet2\tXshimDC\tYshimDC\tZshimDC\tODTpowZ(DipPowZ2)\t0\t1\t0\t0\t0\t1\t0\t0\t0\t0\t0\t0\t0\t0\t0\t0\t0\t0\trMOTdelta(-(rMOTstirDetI +stirWidthF/2))\tODTpowBlue(0)\tODTpowXY(DipPowCr2)\tvarWaveP1\tPdet\tAmp688(depumpPow)\trMOTpow6\tODTpowX(DipPowX2)\tfreq\tHeatingAmp\t0\tSine\tDetuning\tDoppCoolDetF\tsingleFreqDet + 20\tSFCoolT*1000\tDetuning\tDoppCoolStirDet\tsingleFreqStirDet + 20\tSFcoolT*1000\tBlueBN\tBlueLaserProbeBN\tPixisPos(TOF)\tCycle Wait for Move\r\nramp Trap\t\tRamp\t0\trampT\t1\t1\t1\t1\t1\t1\t0\t0\t1\t1\t0\t0\t0\t1\t0\t0\t0\t1\t0\t0\t0\t0\t0\t0\t10u\t0\t1\t0\t0\t0\t1\t1\t0\tplus_zman\tminus_zman\tcompensation\trMOTcurrF\trMOTpow3\tcombAmplitude(combWidthF)\trMOTdelta(-(rMOTbroadDetuningF +combWidthF/2))\tODTpowHLat(DipPowHLat)\t0\t0\t0\t0\t0\t0\t1\t1\tbMOTdelta(MOTdetuning)\tbMOTpow(0.5)\tProbePow\tPdet2\tXshimDC\tYshimDC\tZshimDC\tSinRamp(t,(ODTpowZ(DipPowZ)+ODTpowZ(DipPowZ2))/2,(ODTpowZ(DipPowZ2)-ODTpowZ(DipPowZ))/2,1/(2*rampT),pi/2)\t0\t1\t0\t0\t0\t1\t0\t0\t0\t0\t0\t0\t0\t0\t0\t0\t0\t0\trMOTdelta(-(rMOTstirDetI +stirWidthF/2))\tODTpowBlue(0)\tSinRamp(t,(ODTpowXY(DipPowCr)+ODTpowXY(DipPowCr2))/2,(ODTpowXY(DipPowCr2)-ODTpowXY(DipPowCr))/2,1/(2*rampT),pi/2)\tvarWaveP1\tPdet\tAmp688(depumpPow)\trMOTpow6\tSinRamp(t,(ODTpowX(DipPowX)+ODTpowX(DipPowX2))/2,(ODTpowX(DipPowX2)-ODTpowX(DipPowX))/2,1/(2*rampT),pi/2)\tfreq\tHeatingAmp\t0\tSine\tDetuning\tsingleFreqDetF\tsingleFreqDet + 20\tSFCoolT*1000\tDetuning\tsingleFreqStirDetF\tsingleFreqStirDet + 20\tSFcoolT*1000\tBlueBN\tBlueLaserProbeBN\tPixisPos(TOF)\tCycle Wait for Move\r\nhold\t\tRamp\t0\t.5\t1\t1\t1\t1\t1\t1\t0\t0\t1\t1\t0\t0\t0\t1\t0\t0\t0\t1\t0\t0\t0\t0\t0\t0\t0\t0\t1\t0\t0\t0\t1\t1\t0\tplus_zman\tminus_zman\tcompensation\trMOTcurrF\trMOTpow4\tcombAmplitude(combWidthF)\trMOTdelta(-(rMOTbroadDetuningF +combWidthF/2))\tODTpowHLat(DipPowHLat)\t0\t0\t0\t0\t1\t0\t1\t1\tbMOTdelta(MOTdetuning)\tbMOTpow(0.5)\tProbePow\tPdet2\tXshimDC\tYshimDC\tZshimDC\tODTpowZ(DipPowZ)\t0\t1\t0\t0\t0\t1\t0\t0\t0\t0\t0\t0\t0\t0\t0\t0\t0\t0\trMOTdelta(-(rMOTstirDetI +stirWidthF/2))\tODTpowBlue(0)\tODTpowXY(DipPowCr)\tvarWaveP1\tPdet\tAmp688(depumpPow)\trMOTpow6\tODTpowX(DipPowX)\tfreq\tHeatingAmp\t0\tSine\tDetuning\tDoppCoolDetF\tsingleFreqDet + 20\tSFCoolT*1000\tDetuning\tDoppCoolStirDet\tsingleFreqStirDet + 20\tSFcoolT*1000\tBlueBN\tBlueLaserProbeBN\tPixisPos(TOF)\tCycle Wait for Move\r\nDoppler Cool1\t\tRamp\t0\tdopCoolT\t1\t1\t1\t1\t1\t1\t0\t0\t1\t1\t1\t0\t0\t1\t0\t0\t0\t1\t0\t0\t0\t0\t0\t0\t10u\t0\t1\t0\t0\t0\t1\t1\t1\tplus_zman\tminus_zman\tcompensation\trMOTcurrF\tDoppCoolPow\tcombAmplitude(combWidthF)\trMOTdelta(-(rMOTbroadDetuningF +combWidthF/2))\tODTpowHLat(DipPowHLat)\t0\t0\t0\t0\t1\t0\t1\t1\tbMOTdelta(MOTdetuning)\tbMOTpow(0.5)\tProbePow\tPdet2\tXshimDC\tYshimDC\tZshimDC\tODTpowZ(DipPowZ)\t0\t1\t0\t0\t0\t1\t0\t0\t0\t0\t0\t0\t0\t0\t0\t0\t0\t0\trMOTdelta(-(rMOTstirDetI +stirWidthF/2))\tODTpowBlue(0)\tODTpowXY(DipPowCr)\tvarWaveP1\tPdet\tAmp688(depumpPow)\tDoppStirPow\tODTpowX(DipPowX2)\tfreq\tHeatingAmp\t0\tSine\tDetuning\tDoppCoolDet\tsingleFreqDet + 20\tSFCoolT*1000\tDetuning\tDoppCoolStirDet\tsingleFreqStirDet + 20\tSFcoolT*1000\tBlueBN\tBlueLaserProbeBN\tPixisPos(TOF)\tCycle Wait for Move\r\nDoppler Cool2\t\tRamp\t0\tdopCoolT\t1\t1\t1\t1\t1\t1\t0\t0\t1\t1\t1\t0\t0\t1\t0\t0\t0\t1\t0\t0\t0\t0\t0\t0\t10u\t0\t1\t0\t0\t0\t1\t1\t1\tplus_zman\tminus_zman\tcompensation\trMOTcurrF\trMOTpow5\tcombAmplitude(combWidthF)\trMOTdelta(-(rMOTbroadDetuningF +combWidthF/2))\tODTpowHLat(DipPowHLat)\t0\t0\t0\t0\t1\t0\t1\t1\tbMOTdelta(MOTdetuning)\tbMOTpow(0.5)\tProbePow\tPdet2\tXshimDC\tYshimDC\tZshimDC\tODTpowZ(DipPowZ)\t0\t1\t0\t0\t0\t1\t0\t0\t0\t0\t0\t0\t0\t0\t0\t0\t0\t0\trMOTdelta(-(rMOTstirDetI +stirWidthF/2))\tODTpowBlue(0)\tODTpowXY(DipPowCr)\tvarWaveP1\tPdet\tAmp688(depumpPow)\trMOTpow6\tODTpowX(DipPowX2)\tfreq\tHeatingAmp\t0\tSine\tRamp\tDoppCoolDet\tDoppCoolDet-DoppCoolSweep\tdopCoolT*1000\tDetuning\tDoppCoolStirDet\tsingleFreqStirDet + 20\tSFcoolT*1000\tBlueBN\tBlueLaserProbeBN\tPixisPos(TOF)\tCycle Wait for Move\r\nDoppler Cool3\t\tRamp\t0\tdopCoolT\t1\t1\t1\t1\t1\t1\t0\t0\t1\t1\t1\t0\t0\t1\t0\t0\t0\t1\t0\t0\t0\t0\t0\t0\t10u\t0\t1\t0\t0\t0\t1\t1\t1\tplus_zman\tminus_zman\tcompensation\trMOTcurrF\tLineRamp(f,rMOTpow4,rMOTpow5)\tcombAmplitude(combWidthF)\trMOTdelta(-(rMOTbroadDetuningF +combWidthF/2))\tODTpowHLat(DipPowHLat)\t0\t0\t0\t0\t1\t0\t1\t1\tbMOTdelta(MOTdetuning)\tbMOTpow(0.5)\tProbePow\tPdet2\tXshimDC\tYshimDC\tZshimDC\tODTpowZ(DipPowZ)\t0\t1\t0\t0\t0\t1\t0\t0\t0\t0\t0\t0\t0\t0\t0\t0\t0\t0\trMOTdelta(-(rMOTstirDetI +stirWidthF/2))\tODTpowBlue(0)\tODTpowXY(DipPowCr)\tvarWaveP1\tPdet\tAmp688(depumpPow)\tLineRamp(f,rMOTpow4,rMOTpow5)\tODTpowX(DipPowX2)\tfreq\tHeatingAmp\t0\tSine\tDetuning\tDoppCoolDet-DoppCoolSweep\tDoppCoolDet-DoppCoolSweep\tdopCoolT*1000\tDetuning\tDoppCoolStirDet\tsingleFreqStirDet + 20\tSFcoolT*1000\tBlueBN\tBlueLaserProbeBN\tPixisPos(TOF)\tCycle Wait for Move\r\nhold\t\tRamp\t0\t2\t1\t1\t0\t0\t0\t0\t0\t0\t1\t1\t0\t0\t0\t1\t0\t0\t0\t1\t0\t0\t0\t0\t0\t0\t0\t0\t1\t0\t0\t0\t1\t1\t0\tplus_zman\tminus_zman\tcompensation\trMOTcurrF\trMOTpow4\tcombAmplitude(combWidthF)\trMOTdelta(-(rMOTbroadDetuningF +combWidthF/2))\tODTpowHLat(DipPowHLat)\t0\t0\t0\t0\t0\t0\t1\t1\tbMOTdelta(MOTdetuning)\tbMOTpow(0.5)\tProbePow\tPdet2\tXshim\tYshim\tZshimVar\tODTpowZ(DipPowZ)\t0\t1\t0\t0\t0\t1\t0\t0\t0\t0\t0\t0\t0\t0\t0\t0\t0\t0\trMOTdelta(-(rMOTstirDetI +stirWidthF/2))\tODTpowBlue(0)\tODTpowXY(DipPowCr2)\tvarWaveP1\tPdet\tAmp688(depumpPow)\trMOTpow4\tLineRamp(f, ODTpowX(DipPowX), ODTpowX(DipPowX2))\tfreq\tHeatingAmp\t0\tSine\tDetuning\tDoppCoolDet-DoppCoolSweep\tDoppCoolDet-DoppCoolSweep\tdopCoolT*1000\tDetuning\tDoppCoolStirDet\tsingleFreqStirDet + 20\tSFcoolT*1000\tBlueBN\tBlueLaserProbeBN\tPixisPos(TOF)\tCycle Wait for Move\r\nhold\t\tRamp\t0\tholdT\t1\t1\t0\t0\t0\t0\t0\t0\t1\t1\t0\t0\t0\t1\t0\t0\t0\t1\t0\t0\t0\t0\t0\t0\t0\t0\t1\t0\t0\t0\t1\t1\t0\tplus_zman\tminus_zman\tcompensation\trMOTcurrF\trMOTpow4\tcombAmplitude(combWidthF)\trMOTdelta(-(rMOTbroadDetuningF +combWidthF/2))\tODTpowHLat(DipPowHLat2)\t0\t0\t0\t0\t0\t0\t1\t1\tbMOTdelta(MOTdetuning)\tbMOTpow(0.5)\tProbePow\tPdet2\tXshim\tYshim\tZshimVar\tODTpowZ(DipPowZ)\t0\t1\t0\t0\t1\t1\t0\t0\t0\t0\t0\t0\t0\t0\t0\t0\t0\t0\trMOTdelta(-(rMOTstirDetI +stirWidthF/2))\tODTpowBlue(0)\tODTpowXY(DipPowCr)\tvarWaveP1\tPdet\tAmp688(depumpPow)\trMOTpow4\tODTpowX(DipPowX)\tfreq\tHeatingAmp\t0\tSine\tDetuning\tDoppCoolDet-DoppCoolSweep\tDoppCoolDet-DoppCoolSweep\tdopCoolT*1000\tDetuning\tDoppCoolStirDet\tsingleFreqStirDet + 20\tSFcoolT*1000\tBlueBN\tBlueLaserProbeBN\tPixisPos(TOF)\tCycle Wait for Move\r\ndrop HTrap\t\tRamp\t0\t.03\t1\t1\t1\t1\t1\t1\t0\t0\t1\t1\t0\t0\t0\t1\t0\t0\t0\t1\t0\t0\t0\t0\t0\t0\t0\t0\t1\t0\t0\t0\t1\t1\t0\tplus_zman\tminus_zman\tcompensation\trMOTcurrF\trMOTpow3\tcombAmplitude(combWidthF)\trMOTdelta(-(rMOTbroadDetuningF +combWidthF/2))\tODTpowHLat(DipPowHLat)\t0\t0\t0\t0\t0\t0\t1\t1\tbMOTdelta(MOTdetuning)\tbMOTpow(0.5)\tProbePow\tPdet2\tXshim\tYshim\tZshimVar\tODTpowZ(DipPowZ)\t0\t1\t0\t0\t0\t1\t0\t0\t0\t0\t0\t0\t0\t0\t0\t0\t0\t0\trMOTdelta(-(rMOTstirDetI +stirWidthF/2))\tODTpowBlue(0)\tODTpowXY(DipPowCr)\tvarWaveP1\tPdet\tAmp688(depumpPow)\trMOTpow3\tODTpowX(DipPowX)\tfreq\tHeatingAmp\t0\tSine\tDetuning\tsingleFreqDet\tDoppCoolDet-DoppCoolSweep\tdopCoolT*1000\tDetuning\tsingleFreqStirDet + 20\tsingleFreqStirDet + 20\tSFcoolT*1000\tBlueBN\tBlueLaserProbeBN\tPixisPos(TOF)\tCycle Wait for Move\r\nmodulate\t\tRamp\t0\t3m\t1\t1\t1\t1\t1\t1\t0\t0\t1\t1\t0\t0\t0\t1\t0\t0\t0\t1\t0\t0\t0\t0\t0\t0\t0\t0\t1\t0\t0\t0\t1\t1\t0\tplus_zman\tminus_zman\tcompensation\trMOTcurrF\trMOTpow3\tcombAmplitude(combWidthF)\trMOTdelta(-(rMOTbroadDetuningF +combWidthF/2))\tODTpowHLat(DipPowHLat)\t0\t0\t0\t0\t0\t0\t1\t1\tbMOTdelta(MOTdetuning)\tbMOTpow(0.5)\tProbePow\tPdet2\tXshim\tYshim\tZshimVar\tODTpowZ(DipPowZ)\t0\t1\t0\t0\t0\t1\t0\t0\t0\t0\t0\t0\t0\t0\t0\t0\t0\t0\trMOTdelta(-(rMOTstirDetI +stirWidthF/2))\tODTpowBlue(0)\tODTpowXY(DipPowCr)\tvarWaveP1\tPdet\tAmp688(depumpPow)\trMOTpow3\tODTpowX(DipPowX)\tfreq\tHeatingAmp\t0\tSine\tDetuning\tsingleFreqDet\tDoppCoolDet-DoppCoolSweep\tdopCoolT*1000\tDetuning\tsingleFreqStirDet + 20\tsingleFreqStirDet + 20\tSFcoolT*1000\tBlueBN\tBlueLaserProbeBN\tPixisPos(TOF)\tCycle Wait for Move\r\nEvaporation\t\tRamp\tevapOn\ttEvap1\t1\t1\t1\t1\t1\t1\t0\t0\t1\t1\t0\t0\t0\t1\t0\t0\t0\t1\t0\t0\t0\t0\t0\t0\t1m\t0\t1\t0\t0\t0\t1\t1\t0\tplus_zman\tminus_zman\tcompensation\trMOTcurrF\trMOTpow3\tcombAmplitude(combWidthF)\trMOTdelta(-(rMOTbroadDetuningF +combWidthF/2))\tODTpowHLat(DipPowHLat)\t0\t0\t0\t0\t0\t0\t1\t1\tbMOTdelta(MOTdetuning)\tbMOTpow(0.5)\tProbePow\tPdet2\tXshim\tYshim\tZshimVar\tLineRamp(f,ODTpowZ(DipPowZ2),ODTpowZ(DipPowZ3))\t0\t1\t0\t0\t0\t1\t0\t0\t0\t0\t0\t0\t0\t0\t0\t0\t0\t0\trMOTdelta(-(rMOTstirDetI +stirWidthF/2))\tODTpowBlue(0)\tExpRamp2(t,0,ODTpowXY(DipPowCr2),ODTpowXY(DipPowCr3),tau)\tvarWaveP1\tPdet\tAmp688(depumpPow)\trMOTpow3\tExpRamp2(t,0,ODTpowX(DipPowX2),ODTpowX(DipPowX3),tau)\tfreq\tHeatingAmp\t0\tSine\tDetuning\tsingleFreqDet\tDoppCoolDet-DoppCoolSweep\tdopCoolT*1000\tDetuning\tsingleFreqStirDet + 20\tsingleFreqStirDet + 20\tSFcoolT*1000\tBlueBN\tBlueLaserProbeBN\tPixisPos(TOF)\tCycle Wait for Move\r\nlattice ramp\t\tRamp\t0\t10m\t1\t1\t1\t0\t1\t1\t0\t0\t1\t1\t0\t0\t0\t1\t0\t0\t0\t1\t0\t0\t0\t0\t0\t0\t0\t0\t1\t0\t0\t0\t1\t1\t0\tplus_zman\tminus_zman\tcompensation\trMOTcurrF\trMOTpow3\tcombAmplitude(combWidthF)\trMOTdelta(-(rMOTbroadDetuningF +combWidthF/2))\tODTpowHLat(DipPowHLat)\t0\t0\t0\t0\t0\t0\t1\t1\tbMOTdelta(MOTdetuning)\tbMOTpow(0.5)\tProbePow\tPdet2\tXshim\tYshim\tZshimVar\tODTpowZ(DipPowZ3)\t0\t1\t0\t0\t1\t0\t0\t0\t0\t0\t0\t0\t0\t0\t0\t0\t0\t0\trMOTdelta(-(rMOTstirDetI +stirWidthF/2))\tODTpowBlue(BlueDipPow)\tExpFinal(tEvap1,ODTpowXY(DipPowCr2),ODTpowXY(DipPowCr3),tau)\tvarWaveP2\tPdet\tAmp688(depumpPow)\trMOTpow3\tExpFinal(tEvap1,ODTpowX(DipPowX2),ODTpowX(DipPowX3),tau)\tfreq\tHeatingAmp\t0\tSine\tDetuning\tsingleFreqDet\tDoppCoolDet-DoppCoolSweep\tdopCoolT*1000\tDetuning\tsingleFreqStirDet + 20\tsingleFreqStirDet + 20\tSFcoolT*1000\tBlueBN\tBlueLaserProbeBN\tPixisPos(TOF)\tCycle Wait for Move\r\nbox ramp up\t\tRamp\t0\t1\t1\t1\t1\t1\t1\t1\t0\t0\t1\t1\t0\t0\t0\t1\t0\t0\t0\t1\t0\t0\t0\t0\t0\t0\t10m\t0\t1\t0\t0\t0\t1\t1\t0\tplus_zman\tminus_zman\tcompensation\trMOTcurrF\trMOTpow3\tcombAmplitude(combWidthF)\trMOTdelta(-(rMOTbroadDetuningF +combWidthF/2))\tODTpowHLat(DipPowHLat)\t0\t0\t0\t0\t0\t0\t1\t1\tbMOTdelta(MOTdetuning)\tbMOTpow(0.5)\tProbePow\tPdet2\tXshim\tYshim\tZshimVar\tODTpowZ(DipPowZ3)\t0\t1\t0\t0\t1\t0\t0\t0\t0\t0\t0\t0\t0\t0\t0\t0\t0\t0\trMOTdelta(-(rMOTstirDetI +stirWidthF/2))\tSinRamp(t,(ODTpowBlue(BlueDipPow)+ODTpowBlue(0))/2,(ODTpowBlue(BlueDipPow)-ODTpowBlue(0))/2,1/(2*1),3*pi/2)\tExpFinal(tEvap1,ODTpowXY(DipPowCr2),ODTpowXY(DipPowCr3),tau)\tvarWaveP1\tPdet\tAmp688(depumpPow)\trMOTpow3\tExpFinal(tEvap1,ODTpowX(DipPowX2),ODTpowX(DipPowX3),tau)\tfreq\tHeatingAmp\t0\tSine\tDetuning\tsingleFreqDet\tDoppCoolDet-DoppCoolSweep\tdopCoolT*1000\tDetuning\tsingleFreqStirDet + 20\tsingleFreqStirDet + 20\tSFcoolT*1000\tBlueBN\tBlueLaserProbeBN\tPixisPos(TOF)\tCycle Wait for Move\r\npost evap hold\t\tRamp\t1\t20m\t1\t1\t1\t1\t1\t1\t0\t0\t1\t1\t0\t0\t0\t1\t0\t0\t0\t1\t0\t0\t0\t0\t0\t0\t0\t0\t1\t0\t0\t0\t1\t1\t0\tplus_zman\tminus_zman\tcompensation\trMOTcurrF\trMOTpow3\tcombAmplitude(combWidthF)\trMOTdelta(-(rMOTbroadDetuningF +combWidthF/2))\tODTpowHLat(DipPowHLat2)\t0\t0\t0\t0\t0\t0\t1\t1\tbMOTdelta(MOTdetuning)\tbMOTpow(0.5)\tProbePow\tPdet2\tXshim\tYshim\tZshimVar\tODTpowZ(DipPowZ3)\t0\t1\t0\t0\t1\t0\t0\t0\t0\t0\t0\t0\t0\t0\t0\t0\t0\t0\trMOTdelta(-(rMOTstirDetI +stirWidthF/2))\tODTpowBlue(BlueDipPow)\tExpFinal(tEvap1,ODTpowXY(DipPowCr2),ODTpowXY(DipPowCr3),tau)\tvarWaveP1\tPdet\tAmp688(depumpPow)\trMOTpow3\tExpFinal(tEvap1,ODTpowX(DipPowX2),ODTpowX(DipPowX3),tau)\tfreq\tHeatingAmp\t0\tSine\tDetuning\tsingleFreqDet\tDoppCoolDet-DoppCoolSweep\tdopCoolT*1000\tDetuning\tsingleFreqStirDet + 20\tsingleFreqStirDet + 20\tSFcoolT*1000\tBlueBN\tBlueLaserProbeBN\tPixisPos(TOF)\tCycle Wait for Move\r\npost evap\t\tRamp\t1\tpulseLatT\t1\t1\t1\t1\t1\t1\t0\t0\t1\t1\t0\t0\t0\t1\t0\t0\t0\t1\t0\t0\t0\t0\t0\t0\t0\t0\t1\t0\t0\t0\t1\t1\t0\tplus_zman\tminus_zman\tcompensation\trMOTcurrF\trMOTpow3\tcombAmplitude(combWidthF)\trMOTdelta(-(rMOTbroadDetuningF +combWidthF/2))\tODTpowHLat(DipPowHLat2)\t0\t0\t0\t0\t0\t0\t1\t1\tbMOTdelta(MOTdetuning)\tbMOTpow(0.5)\tProbePow\tPdet2\tXshim\tYshim\tZshimVar\tODTpowZ(DipPowZ3)\t0\t1\t0\t0\t1\t1\t0\t0\t0\t0\t0\t0\t0\t0\t0\t0\t0\t0\trMOTdelta(-(rMOTstirDetI +stirWidthF/2))\tODTpowBlue(BlueDipPow)\tExpFinal(tEvap1,ODTpowXY(DipPowCr2),ODTpowXY(DipPowCr3),tau)\tvarWaveP1\tPdet\tAmp688(depumpPow)\trMOTpow3\tExpFinal(tEvap1,ODTpowX(DipPowX2),ODTpowX(DipPowX3),tau)\tfreq\tHeatingAmp\t0\tSine\tDetuning\tsingleFreqDet\tDoppCoolDet-DoppCoolSweep\tdopCoolT*1000\tDetuning\tsingleFreqStirDet + 20\tsingleFreqStirDet + 20\tSFcoolT*1000\tBlueBN\tBlueLaserProbeBN\tPixisPos(TOF)\tCycle Wait for Move\r\npost evap hold\t\tRamp\t0\t2*rampLatT\t1\t1\t1\t1\t1\t1\t0\t0\t1\t1\t0\t0\t0\t1\t0\t0\t0\t1\t0\t0\t0\t0\t0\t0\t0\t0\t1\t0\t0\t0\t1\t1\t0\tplus_zman\tminus_zman\tcompensation\trMOTcurrF\trMOTpow3\tcombAmplitude(combWidthF)\trMOTdelta(-(rMOTbroadDetuningF +combWidthF/2))\tODTpowHLat(DipPowHLat)\t0\t0\t0\t0\t0\t0\t1\t1\tbMOTdelta(MOTdetuning)\tbMOTpow(0.5)\tProbePow\tPdet2\tXshim\tYshim\tZshimVar\tODTpowZ(DipPowZ3)\t0\t1\t0\t0\t1\t0\t0\t0\t0\t0\t0\t0\t0\t0\t0\t0\t0\t0\trMOTdelta(-(rMOTstirDetI +stirWidthF/2))\tODTpowBlue(BlueDipPow)\tExpFinal(tEvap1,ODTpowXY(DipPowCr2),ODTpowXY(DipPowCr3),tau)\tvarWaveP1\tPdet\tAmp688(depumpPow)\trMOTpow3\tExpFinal(tEvap1,ODTpowX(DipPowX2),ODTpowX(DipPowX3),tau)\tfreq\tHeatingAmp\t0\tSine\tDetuning\tsingleFreqDet\tDoppCoolDet-DoppCoolSweep\tdopCoolT*1000\tDetuning\tsingleFreqStirDet + 20\tsingleFreqStirDet + 20\tSFcoolT*1000\tBlueBN\tBlueLaserProbeBN\tPixisPos(TOF)\tCycle Wait for Move\r\nlattice rampup\t\tRamp\t0\trampLatT\t1\t1\t1\t1\t1\t1\t0\t0\t1\t1\t0\t0\t0\t1\t0\t0\t0\t1\t0\t0\t0\t0\t0\t0\t10u\t0\t1\t0\t0\t0\t1\t1\t0\tplus_zman\tminus_zman\tcompensation\trMOTcurrF\trMOTpow3\tcombAmplitude(combWidthF)\trMOTdelta(-(rMOTbroadDetuningF +combWidthF/2))\tSinRamp(t,(ODTpowHLat(DipPowHLat)+ODTpowHLat(DipPowHLat2))/2,(ODTpowHLat(DipPowHLat)-ODTpowHLat(DipPowHLat2))/2,1/(2*rampLatT), pi/2)\t0\t0\t0\t0\t0\t0\t1\t1\tbMOTdelta(MOTdetuning)\tbMOTpow(0.5)\tProbePow\tPdet2\tXshim\tYshim\tZshimVar\tSinRamp(t,(ODTpowZ(DipPowZ3)+ODTpowZ(DipPowZLat))/2, (ODTpowZ(DipPowZ3)-ODTpowZ(DipPowZLat))/2, 1/(2*rampLatT), pi/2)\t0\t1\t0\t0\t1\t0\t0\t0\t0\t0\t0\t0\t0\t0\t0\t0\t0\t0\trMOTdelta(-(rMOTstirDetI +stirWidthF/2))\tODTpowBlue(0)\tExpFinal(tEvap1,ODTpowXY(DipPowCr2),ODTpowXY(DipPowCr3),tau)\tLineRamp(f,varWaveP1,varWaveP2)\tPdet\tAmp688(depumpPow)\trMOTpow3\tExpFinal(tEvap1,ODTpowX(DipPowX2),ODTpowX(DipPowX3),tau)\tfreq\tHeatingAmp\t0\tSine\tDetuning\tsingleFreqDet\tDoppCoolDet-DoppCoolSweep\tdopCoolT*1000\tDetuning\tsingleFreqStirDet + 20\tsingleFreqStirDet + 20\tSFcoolT*1000\tBlueBN\tBlueLaserProbeBN\tPixisPos(TOF)\tCycle Wait for Move\r\nODT rampdown\t\tRamp\t0\trampLatT\t1\t1\t1\t1\t1\t1\t0\t0\t1\t1\t0\t0\t0\t1\t0\t0\t0\t1\t0\t0\t0\t0\t0\t0\t1m\t0\t1\t0\t0\t0\t1\t1\t0\tplus_zman\tminus_zman\tcompensation\trMOTcurrF\trMOTpow3\tcombAmplitude(combWidthF)\trMOTdelta(-(rMOTbroadDetuningF +combWidthF/2))\tODTpowHLat(DipPowHLat2)\t0\t0\t0\t0\t0\t0\t1\t1\tbMOTdelta(MOTdetuning)\tbMOTpow(0.5)\tProbePow\tPdet2\tXshim\tYshim\tZshimVar\tODTpowZ(DipPowZLat)\t0\t1\t0\t0\t1\t1\t0\t0\t0\t0\t0\t0\t0\t0\t0\t0\t0\t0\trMOTdelta(-(rMOTstirDetI +stirWidthF/2))\tODTpowBlue(0)\tSinRamp(t,(ExpFinal(tEvap1,ODTpowXY(DipPowCr2),ODTpowXY(DipPowCr3),tau)+ODTpowXY(0))/2,(ODTpowXY(0)-ExpFinal(tEvap1,ODTpowXY(DipPowCr2),ODTpowXY(DipPowCr3),tau))/2,1/(2*rampLatT),3*pi/2)\tvarWaveP2\tPdet\tAmp688(depumpPow)\trMOTpow3\tSinRamp(t,(ExpFinal(tEvap1,ODTpowX(DipPowX2),ODTpowX(DipPowX3),tau)+ODTpowX(0))/2,(ODTpowX(0)-ExpFinal(tEvap1,ODTpowX(DipPowX2),ODTpowX(DipPowX3),tau))/2,1/(2*rampLatT),3*pi/2)\tfreq\tHeatingAmp\t0\tSine\tDetuning\tsingleFreqDet\tDoppCoolDet-DoppCoolSweep\tdopCoolT*1000\tDetuning\tsingleFreqStirDet + 20\tsingleFreqStirDet + 20\tSFcoolT*1000\tBlueBN\tBlueLaserProbeBN\tPixisPos(TOF)\tCycle Wait for Move\r\nlattice hold\t\tRamp\t0\t100m\t1\t1\t1\t1\t1\t1\t0\t0\t1\t1\t0\t0\t0\t1\t0\t0\t0\t1\t0\t0\t0\t0\t0\t0\t1m\t0\t1\t0\t0\t0\t1\t1\t0\tplus_zman\tminus_zman\tcompensation\t